vi "garabato FM.vi"() -> ()   [LabVIEW 2019]
uses:
  <vilib>/Analysis/3filter.llb/Filter Passband Type.ctl
  <vilib>/Waveform/WDTOps.llb/WDT Get Waveform Time Array DBL.vi
  <vilib>/measure/maspectr.llb/FFT Power Spectrum and PSD for 1 Chan.vi
  <vilib>/express/express analysis/Spectral/Block/exnSpectralBlock spectral measurements peak poly.vi
  <vilib>/express/express analysis/Spectral/Block/exnSpectralBlock spectral measurements peak WFM.vi
  <vilib>/Analysis/3filter.llb/Butterworth Filter (DBL).vi
  <vilib>/express/express analysis/Spectral/XNode/ExpressSpectralMeasurementsBlockNode.xnode
  <vilib>/measure/NI_MABase.lvlib
  <vilib>/Analysis/NI_AALPro.lvlib
  <vilib>/measure/NI_MAPro.lvlib
  <vilib>/Analysis/NI_AALBase.lvlib
panel:
  in  "Volumen":dbl(slide)=4045.8015267175574 scale=0.0..10000.0
  in  "Boolean":bool
  in  "stop":bool
  out "Espectro Recuperado":cluster{"f0":dbl, "df":dbl, "magnitude":dbl[]}(graph)={"f0"=0.0, "df"=0.0459375, "magnitude"=[]}
  out "Señal Recuperada":waveform(dbl)(graph)={"t0"=timestamp(0 s since 1904-01-01), "dt"=2.2675736961451248e-05, "Y"=[]}
  out "dt":dbl=1.0416666666666666e-05
  out "Frecuencia del mensaje":dbl=2548.361796429108
  in  "Datos del mensaje":T1={"Frecuencia del mensaje"=2548.361796429108, "Amplitud del mensaje"=3.139081873854861, "Fase del mensaje"=0.0} {"Fase del mensaje" scale=0.0..90.0; "Amplitud del mensaje" scale=0.0..10.0; "Frecuencia del mensaje" scale=0.0..3500.0}
  in  "?":T2(tab)=enum."Señal detectada"
  out "Mensaje  en frecuencia":cluster{"f0":dbl, "df":dbl, "magnitude":dbl[]}(graph)={"f0"=0.0, "df"=0.1, "magnitude"=[]}
  out "Mensaje en tiempo":waveform(dbl)(graph)={"t0"=timestamp(0 s since 1904-01-01), "dt"=1.0416666666666666e-05, "Y"=[]}
  out "Mensaje modulado en frecuencia":cluster{"f0":dbl, "df":dbl, "magnitude":dbl[]}(graph)={"f0"=0.0, "df"=0.1, "magnitude"=[]}
  out "Mensaje modulado en tiempo":waveform(dbl)(graph)={"t0"=timestamp(0 s since 1904-01-01), "dt"=1.0416666666666666e-05, "Y"=[]}
  out "Delta w":dbl=1700.0
  out "Beta":sgl=0.037777778
  in  "Kf":dbl=1700.0
  out "Señal Detectada":waveform(dbl)(graph)={"t0"=timestamp(0 s since 1904-01-01), "dt"=1.0416666666666666e-05, "Y"=[]}
  out "Espectro Detectado":cluster{"f0":dbl, "df":dbl, "magnitude":dbl[]}(graph)={"f0"=0.0, "df"=0.1, "magnitude"=[]}
  in  "Datos de la portadora":T3={"Frecuencia de la portadora"=45000.0, "Amplitud de la portadora"=7.013349106979103, "Fase de la portadora"=0.0} {"Fase de la portadora" scale=0.0..90.0; "Amplitud de la portadora" scale=0.0..10.0; "Frecuencia de la portadora" scale=0.0..45000.0}
  in  "Muestreo":cluster{"Fs":dbl, "#s":dbl}={"Fs"=1000000.0, "#s"=1000000.0} {"Fs" format="%.2p"}
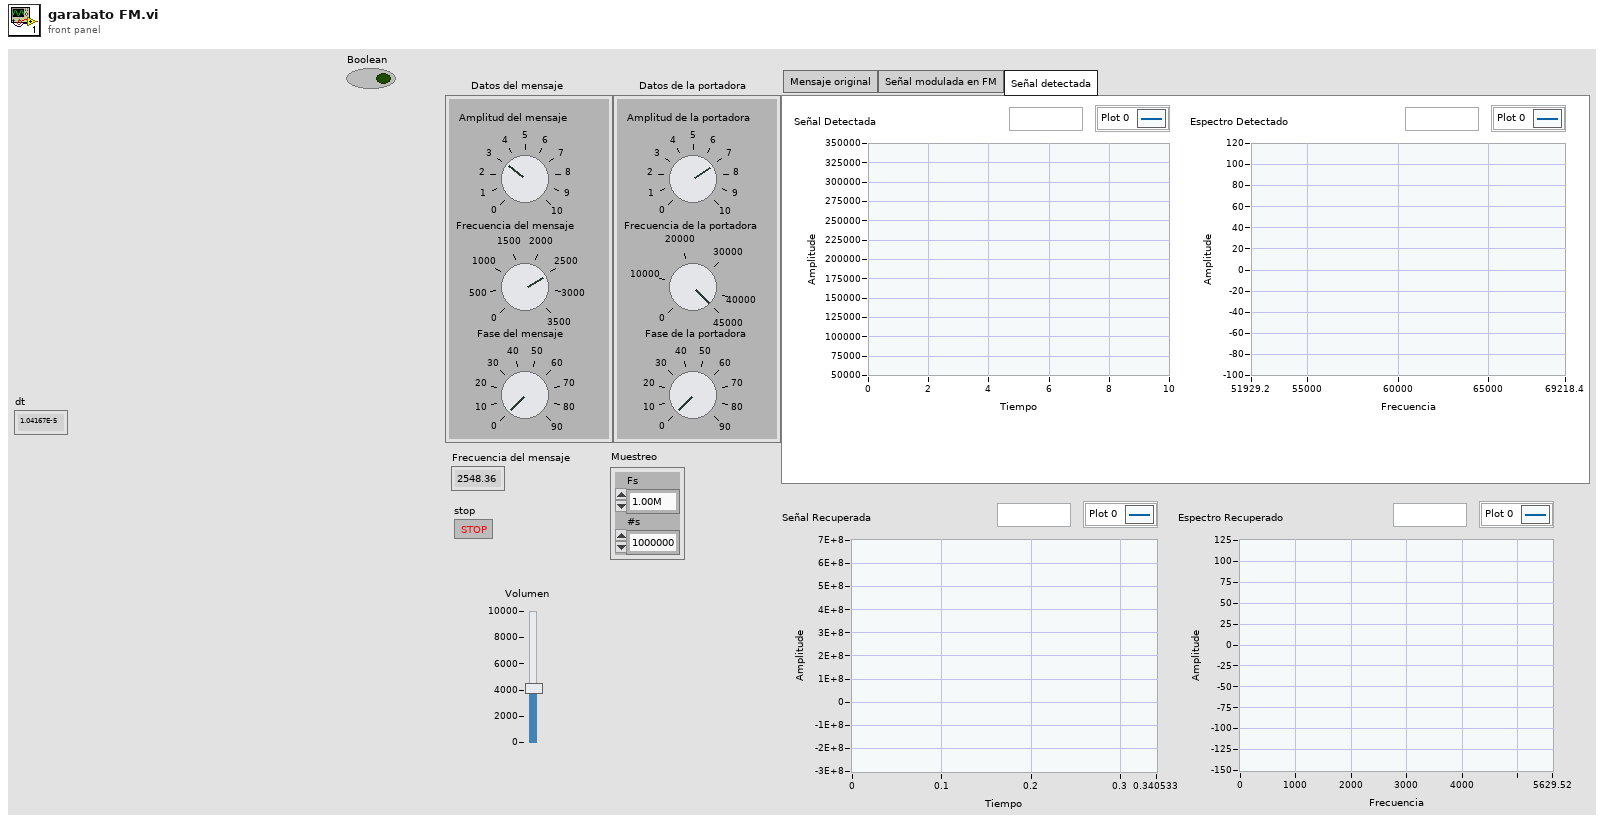
[diagram p1: front panel]
types:
  T1 = cluster{"Frecuencia del mensaje":dbl, "Amplitud del mensaje":dbl, "Fase del mensaje":dbl}
  T2 = enum32{"Mensaje original", "Señal modulada en FM", "Señal detectada"}
  T3 = cluster{"Frecuencia de la portadora":dbl, "Amplitud de la portadora":dbl, "Fase de la portadora":dbl}
  T4 = typedef "NI_AALBase.lvlib/Filter Passband Type.ctl" = enum32{"Lowpass", "Highpass", "Bandpass", "Bandstop"}
  T5 = cluster{"averaging mode":u16, "weighting mode":u16, "number of averages":u32}
  T6 = cluster{"dB On (F)":bool, "unwrap phase (F)":bool, "convert to degree (F)":bool}
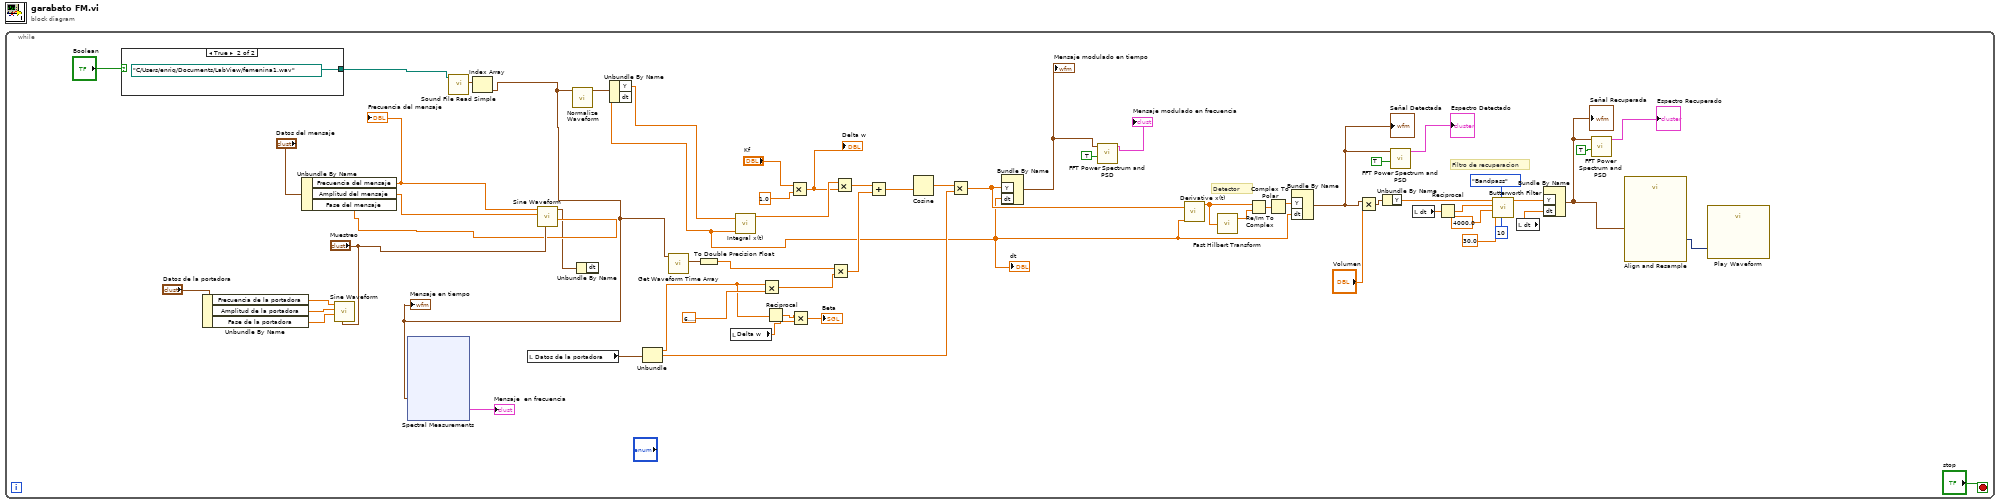
[diagram p0: block diagram]
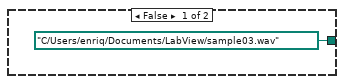
[diagram p2: hidden frame]
diagram:
  n1 = while {
    stop <- "stop" stop-if-true
    # "Filtro de recuperacion"
    # "Detector"
    n2 = case shown="True" "Boolean" {
      tunnel: [path "C:/Users/enriq/Documents/LabView/sample03.wav" ("path") path "C:/Users/enriq/Documents/LabView/femenina1.wav" ("path")] -> w23
      frame False {
      }
      frame True {
      }
    }
    n3 = Unbundle By Name("Datos de la portadora") -> ("Frecuencia de la portadora"=w62:dbl, "Amplitud de la portadora"=w61:dbl, "Fase de la portadora"=w50:dbl)
    n4 = Unbundle By Name("Datos del mensaje") -> ("Frecuencia del mensaje"=w40:dbl, "Amplitud del mensaje"=w39:dbl, "Fase del mensaje"=w38:dbl)
    "Frecuencia del mensaje" <- w40
    n5 = call <vilib>:"Sine Waveform.vi"("sampling info"="Muestreo", "phase"=w50, "amplitude"=w61, "frequency"=w62) -> ()  [unwired: 6 in, 2 out]
    n6 = call <vilib>:"Sound File Read Simple.vi"("path"=w23) -> ("data"=w24:waveform(dbl)[])  [unwired: 7 in, 3 out]
    n7 = Index Array(array=w24) -> (element=w13:waveform(dbl))  [unwired: 1 in]
    "Mensaje en tiempo" <- w13
    n8 = xnode "Spectral Measurements"("Signals"=w13) -> ("FFT - (Peak)"=→"Mensaje  en frecuencia":cluster{"f0":dbl, "df":dbl, "magnitude":dbl[]})  [unwired: 2 in, 3 out]
    n9 = local read "Datos de la portadora"() -> (w58:T3)
    n10 = call <vilib>:"Sine Waveform.vi"("sampling info"="Muestreo", "phase"=w38, "amplitude"=w39, "frequency"=w40) -> ("signal out"=w18:waveform(dbl))  [unwired: 6 in, 1 out]
    n11 = call <vilib>:"Normalize Waveform.vi"("waveform in"=w13) -> ("normalized waveform"=w14:waveform(dbl))  [unwired: 7 in, 3 out]
    n12 = Unbundle By Name(w18) -> ()  [unwired: 1 out]
    n13 = Unbundle By Name(w14) -> ("Y"=w15:dbl[], "dt"=w7:dbl)
    "dt" <- w7
    n14 = Unbundle(w58) -> ("Frecuencia de la portadora"=w25:dbl, "Amplitud de la portadora"=w51:dbl)  [unwired: 1 out]
    n15 = call-poly <vilib>:"Get Waveform Time Array.vi"("waveform in"=w13) -> ("X array"=w59:timestamp[])  [unwired: 9 in, 1 out]
    n16 = To Double Precision Float(number=w59) -> (double precision float=w56:dbl[])
    n17 = local read "Delta w"() -> (w46:dbl)
    n18 = call <vilib>:"Integral x(t).vi"("dt"=w7, "X"=w15) -> ("Integral X"=w63:dbl[])  [unwired: 8 in, 1 out]
    n19 = Multiply(x=w25, y=6.283185307179586) -> (x*y=w48:dbl)
    n20 = Reciprocal(x=w25) -> (1/x=w47:dbl)
    n21 = Multiply(x="Kf", y=1.0) -> (x*y=w45:dbl)
    "Delta w" <- w45
    n22 = Multiply(x=w47, y=w46) -> (x*y=→"Beta":dbl)
    n23 = Multiply(x=w56, y=w48) -> (x*y=w54:dbl[])
    n24 = Multiply(x=w63, y=w45) -> (x*y=w55:dbl[])
    n25 = Add(x=w55, y=w54) -> (x+y=w53:dbl[])
    n26 = Cosine(x=w53) -> (cos(x)=w52:dbl[])
    n27 = Multiply(x=w52, y=w51) -> (x*y=w22:dbl[])
    n28 = Bundle By Name("Y"=w22, "dt"=w7) -> (w21:waveform(dbl))  [unwired: 1 in]
    "Mensaje modulado en tiempo" <- w21
    n29 = call-poly <vilib>:"FFT Power Spectrum and PSD.vi"("dB On (F)"=TRUE, "time signal"=w21) -> ("Power Spectrum / PSD"=→"Mensaje modulado en frecuencia":cluster{"f0":dbl, "df":dbl, "magnitude":dbl[]})  [unwired: 6 in, 3 out]
    n30 = call <vilib>:"Derivative x(t).vi"("dt"=w7, "X"=w22) -> ("dX/dt"=w3:dbl[])  [unwired: 8 in, 1 out]
    n31 = call <vilib>:"Fast Hilbert Transform.vi"("X"=w3) -> ("Hilbert{X}"=w10:dbl[])  [unwired: 1 out]
    n32 = Re/Im To Complex(1:w10, 2:w3) -> (0:w9:cdb[])
    n33 = Complex To Polar(r * e^(i*theta)=w9) -> (r=w8:dbl[])  [unwired: 1 out]
    n34 = Bundle By Name("Y"=w8, "dt"=w7) -> (w5:waveform(dbl))  [unwired: 1 in]
    "Señal Detectada" <- w5
    n35 = Multiply(x=w5, y="Volumen") -> (x*y=w4:waveform(dbl))
    n36 = Unbundle By Name(w4) -> ("Y"=w16:dbl[])
    n37 = call-poly <vilib>:"FFT Power Spectrum and PSD.vi"("dB On (F)"=TRUE, "time signal"=w5) -> ("Power Spectrum / PSD"=→"Espectro Detectado":cluster{"f0":dbl, "df":dbl, "magnitude":dbl[]})  [unwired: 6 in, 3 out]
    n38 = local read "dt"() -> (w31:dbl)
    n39 = Reciprocal(x=w31) -> (1/x=w35:dbl)
    n40 = call-poly <vilib>:"Butterworth Filter.vi"("order"=10, "filter type"=Filter_Passband_Type."Bandpass", "low cutoff freq: fl"=30.0, "high cutoff freq: fh"=4000.0, "sampling freq: fs"=w35, "X"=w16) -> ("Filtered X"=w28:dbl[])  [unwired: 2 in, 1 out]
    n41 = local read "dt"() -> (w32:dbl)
    n42 = Bundle By Name("Y"=w28, "dt"=w32) -> (w2:waveform(dbl))  [unwired: 1 in]
    "Señal Recuperada" <- w2
    n43 = call-poly <vilib>:"FFT Power Spectrum and PSD.vi"("dB On (F)"=TRUE, "time signal"=w2) -> ("Power Spectrum / PSD"=→"Espectro Recuperado":cluster{"f0":dbl, "df":dbl, "magnitude":dbl[]})  [unwired: 6 in, 3 out]
    n44 = call "Align and Resample"("Signals"=w2) -> ("Resampled Signals"=w1:dynamicdata)  [unwired: 8 in, 2 out]
    n45 = call "Play Waveform"("Data"=w1) -> ()  [unwired: 18 in, 1 out]
  }
